vi "UHR-Fleezers Control (host) - 10.3.vi"() -> ()   [LabVIEW 2010] (continued)
        n1173 = Boolean To (0,1)(Boolean="Trap 2 ON") -> (0, 1=w4497:i16)
        n1174 = Select(t=w4497, s="Trap ON/OFF X or Y Amp?", f=w4494) -> (s? t:f=w4492:i16)
        n1175 = Select(t=w4496, s="Trap ON/OFF X or Y Amp?", f=w4494) -> (s? t:f=w4493:i16)
        n1176 = Select(t=w4495, s="Trap ON/OFF X or Y Amp?", f=w4494) -> (s? t:f=w4491:i16)
        n1177 = Select(t=w4494, s="Trap ON/OFF X or Y Amp?", f=w4497) -> (s? t:f=w4489:i16)
        n1178 = Select(t=w4494, s="Trap ON/OFF X or Y Amp?", f=w4496) -> (s? t:f=w4490:i16)
        n1179 = Select(t=w4494, s="Trap ON/OFF X or Y Amp?", f=w4495) -> (s? t:f=w4488:i16)
        n1180 = And(x="All FB On/Off", y="Feedback On/Off") -> (x .and. y?=w4486:cluster{"Set 1":bool, "Set 2":bool})
        n1181 = local read "BD 1 Amplitude 1 (%)"() -> (w4506:dbl)
        n1182 = local read "BD 1 Amplitude 2 (%)"() -> (w4505:dbl)
        n1183 = local read "BD 1 Amplitude 3 (%)"() -> (w4504:dbl)
        n1184 = Unbundle By Name(w4486) -> ("Set 1"=w4481:bool, "Set 2"=w4478:bool)
        n1185 = local read "Y RF Amplitude Limits (%)"() -> (w4474:T16)
        n1186 = local read "X RF Amplitude Limits (%)"() -> (w4475:T16)
        n1187 = local read "BD 2 Amplitude 1 (%)"() -> (w4507:dbl)
        n1188 = local read "BD 2 Amplitude 2 (%)"() -> (w4508:dbl)
        n1189 = local read "BD 2 Amplitude 3 (%)"() -> (w4509:dbl)
        n1190 = And(x="Trap 2 ON", y=w4478) -> (x .and. y?=w4476:bool)
        n1191 = And(x="Trap 1 ON", y=w4481) -> (x .and. y?=w4479:bool)
        n1192 = Multiply(x=w4493, y=w4506) -> (x*y=w4501:dbl)
        n1193 = Multiply(x=w4505, y=w4492) -> (x*y=w4499:dbl)
        n1194 = Multiply(x=w4504, y=w4491) -> (x*y=w4500:dbl)
        n1195 = Multiply(x=w4507, y=w4490) -> (x*y=w4510:dbl)
        n1196 = Multiply(x=w4508, y=w4489) -> (x*y=w4511:dbl)
        n1197 = Multiply(x=w4509, y=w4488) -> (x*y=w4512:dbl)
        n1198 = call "set RF board amplitude - interlace.vi"("Board 2 Amplitude Limits"=w4474, "Board 1 Amplitude Limits"=w4475, "error in"=w4502, "FPGA VI Reference In"=w4503, "Board 2 Amplitude 3 (%)"=w4512, "Board 1 Amplitude 3 (%)"=w4500, "Board 2 Amplitude 2 (%)"=w4511, "Board 2 Amplitude 1 (%)"=w4510, "Board 1 Amplitude 2 (%)"=w4499, "Board 1 Amplitude 1 (%)"=w4501) -> ("error out"=w4483:errorcluster, "FPGA VI Reference Out"=w4484:T19)
        n1199 = xnode "Read/Write Control"("FPGA VI Reference In"=w4484, "error in"=w4483, "FB On/Off Set 1"=w4479, "FB On/Off Set 2"=w4476) -> ("error out"=w4482:errorcluster)  [unwired: 1 out]
      }
      event "Load parameters": Value Change {
        n1200 = event-data() -> ()  [unwired: 7 out]
        n1201 = property on="Saved AOD Raster Scan Parameter Sets" class="Arr (strict)"() -> ("Index Values"=w4582:u32[])  [unwired: 2 in, 2 out]
        n1202 = Index Array(array=w4582, index=0) -> (element=w4579:u32)
        n1203 = local write "Load parameters"(FALSE ("Load parameters")) -> ()
        n1204 = Index Array(array="Saved AOD Raster Scan Parameter Sets", index=w4579) -> (element=w4578:T42)
        n1205 = Unbundle By Name(w4578) -> ("Scan Range AOD (nm) 2"=w4577:dbl, "Step Size AOD (nm) 2"=w4576:dbl, "Scan Speed AOD (nm/s) 2"=w4575:dbl, "Number of scans (AOD) 2"=w4574:u16)
        n1206 = flat-sequence {
          tunnel: w4577 -> [w4585]
          tunnel: w4576 -> [w4584]
          tunnel: w4575 -> [w4583]
          tunnel: w4574 -> [w4586]
          frame #0 {
            n1207 = local write "Scan Speed (nm/s)"(w4583) -> ()
            n1208 = local write "Scan Range (nm)"(w4585) -> ()
            n1209 = local write "Step Size (nm)"(w4584) -> ()
          }
          frame #1 {
            n1210 = property on="Number of F/B Scans (AOD)" class="DigNum (strict)"("Val(Sgnl)"=w4586) -> ()  [unwired: 2 in, 2 out]
          }
        }
      }
      event "Trap 1 (ON/OFF)", "Trap 2 (ON/OFF)": Value Change {
        n1211 = event-data() -> ()  [unwired: 7 out]
        n1212 = property on="Trap 2 ON" class="Bool (strict)"("Val(Sgnl)"="Trap 2 (ON/OFF)") -> ()  [unwired: 2 in, 2 out]
        n1213 = property on="Trap 1 ON" class="Bool (strict)"("Val(Sgnl)"="Trap 1 (ON/OFF)") -> ()  [unwired: 2 in, 2 out]
      }
      event "DIO count 1 (ticks)", "DIO count 2 (ticks)", "DIO count 3 (ticks)", "Interlace", "Number Interlace Sets", "Not-Interlacing Set": Value Change {
        n1214 = event-data() -> ()  [unwired: 7 out]
        n1215 = local read "DIO count 3 (ticks)"() -> (w4599:u32)
        n1216 = local read "DIO count 1 (ticks)"() -> (w4601:u32)
        n1217 = local read "DIO count 2 (ticks)"() -> (w4600:u32)
        n1218 = To Unsigned Byte Integer(number="Not-Interlacing Set") -> (unsigned 8bit integer=w4590:u8)
        n1219 = Add(x=w4590, y=u8 1) -> (x+y=w4594:u8)
        n1220 = xnode "Read/Write Control"("FPGA VI Reference In"=w4605, "error in"=w4603, "DIO count 1 (ticks)"=w4601, "DIO count 2 (ticks)"=w4600, "DIO count 3 (ticks)"=w4599, "Interlace ON/OFF"="Interlace", "Number Interlace Cycles"="Number Interlace Sets", "Interlace Off Parameters"=w4594) -> ("error out"=w4604:errorcluster)  [unwired: 1 out]
        n1221 = Build Array(w4601, w4600, w4599) -> (w4592:u32[])
        n1222 = Split 1D Array(array=w4592, index="Number Interlace Sets") -> (first subarray=w4602:u32[])  [unwired: 1 out]
        n1223 = Index Array(array=w4592, index=w4590) -> (element=w4591:u32)
        n1224 = Add Array Elements(numeric array=w4602) -> (sum=w4596:u32)
        n1225 = Select(t=w4596, s="Interlace", f=w4591) -> (s? t:f=→"Total Counts (ticks)":u32)
      }
      event "Reset Feedback": Value Change {
        n1226 = event-data() -> ()  [unwired: 7 out]
        n1227 = Unbundle By Name("Reset Feedback") -> ("Set 1"=w4747:bool, "Set 2"=w4746:bool)
        n1228 = xnode "Read/Write Control"("FPGA VI Reference In"=w4749, "error in"=w4744, "FB Reset Set 1"=w4747, "FB Reset Set 2"=w4746) -> ("error out"=w4745:errorcluster)  [unwired: 1 out]
      }
      event "PID Gains": Value Change {
        n1229 = event-data() -> ()  [unwired: 7 out]
        n1230 = Unbundle By Name("PID Gains") -> ("Set 1"=w4812:T14, "Set 2"=w4811:T14)
        n1231 = xnode "Read/Write Control"("FPGA VI Reference In"=w4813, "error in"=w4809, "FB Gains Set 1"=w4812, "FB Gains Set 2"=w4811) -> ("error out"=w4810:errorcluster)  [unwired: 1 out]
      }
      event "AI2 to Setpoint", "Setpoints (V)": Value Change {
        n1232 = event-data() -> ()  [unwired: 7 out]
        n1233 = xnode "Read/Write Control"("FPGA VI Reference In"=w4888, "error in"=w4884) -> ("FPGA VI Reference Out"=w4887:T19, "error out"=w4886:errorcluster, "AI2 Y Sum Set 1"=w4895:i16, "AI2 Y Sum Set 2"=w4894:i16)
        n1234 = Cluster To Array(cluster="AI2 to Setpoint") -> (array=w4898:bool[])
        n1235 = local read "AI2 (V)"() -> (w4896:cluster{"Set 1":dbl, "Set 2":dbl})
        n1236 = Or Array Elements(Boolean array=w4898) -> (logical OR=w4899:bool)
        n1237 = Bundle By Name(cluster=w4896, "Set 1"=w4895, "Set 2"=w4894) -> (w4893:cluster{"Set 1":dbl, "Set 2":dbl})
        n1238 = Divide(x=w4893, y=3276.7) -> (x/y=w4892:cluster{"Set 1":dbl, "Set 2":dbl})
        "AI2 (V)" <- w4892
        n1239 = case shown="True" w4899 {
          tunnel: [w4963 w4980] -> w4891
          tunnel: "AI2 to Setpoint" -> [_ w4976]
          tunnel: "Setpoints (V)" -> [w4964 w4979]
          tunnel: w4892 -> [_ w4973]
          frame False {
            n1240 = Multiply(x=3276.7, y=w4964) -> (x*y=w4965:cluster{"Set 1":dbl, "Set 2":dbl})
            n1241 = To Word Integer(number=w4965) -> (16bit integer=w4963:cluster{"Set 1":i16, "Set 2":i16})
          }
          frame True {
            n1242 = Unbundle By Name(w4973) -> ("Set 1"=w4972:dbl, "Set 2"=w4971:dbl)
            n1243 = Unbundle By Name(w4979) -> ("Set 1"=w4978:dbl, "Set 2"=w4977:dbl)
            n1244 = Unbundle By Name(w4976) -> ("Set 1"=w4975:bool, "Set 2"=w4974:bool)
            n1245 = Select(t=w4972, s=w4975, f=w4978) -> (s? t:f=w4970:dbl)
            n1246 = Select(t=w4971, s=w4974, f=w4977) -> (s? t:f=w4969:dbl)
            n1247 = Bundle By Name(cluster=w4979, "Set 1"=w4970, "Set 2"=w4969) -> (w4967:cluster{"Set 1":dbl, "Set 2":dbl})
            n1248 = local write "Setpoints (V)"(w4967) -> ()
            n1249 = Multiply(x=3276.7, y=w4967) -> (x*y=w4968:cluster{"Set 1":dbl, "Set 2":dbl})
            n1250 = To Word Integer(number=w4968) -> (16bit integer=w4980:cluster{"Set 1":i16, "Set 2":i16})
          }
        }
        n1251 = Unbundle By Name(w4891) -> ("Set 1"=w4890:i16, "Set 2"=w4889:i16)
        n1252 = xnode "Read/Write Control"("FPGA VI Reference In"=w4887, "error in"=w4886, "FB Setpoint Set 1"=w4890, "FB Setpoint Set 2"=w4889) -> ("error out"=w4885:errorcluster)  [unwired: 1 out]
      }
      event "Invert GI": Value Change {
        n1253 = event-data() -> ()  [unwired: 7 out]
        n1254 = xnode "Read/Write Control"("FPGA VI Reference In"=w5042, "error in"=w5040, "Invert GI"="Invert GI", "Invert GI 2"="Invert GI") -> ("error out"=w5041:errorcluster)  [unwired: 1 out]
      }
      event "Green FB Setpoint (mV)", "Green FB Gains", "Green FB On/Off", "Current When FB OFF (%)", "Green int current ON count adj": Value Change {
        n1255 = event-data() -> ()  [unwired: 7 out]
        n1256 = local read "Green FB Setpoint (mV)"() -> (w5108:dbl)
        n1257 = local read "Current When FB OFF (%)"() -> (w5111:dbl)
        n1258 = Multiply(x=w5108, y=3.2767) -> (x*y=w5107:dbl)
        n1259 = Multiply(x=w5111, y=655.35) -> (x*y=w5112:dbl)
        n1260 = To Unsigned Word Integer(number=w5112) -> (unsigned 16bit integer=w5110:u16)
        n1261 = local read "Green int current ON count adj"() -> (w5115:u32)
        n1262 = local read "Green FB Gains"() -> (w5114:T14)
        n1263 = local read "Green Laser ON/Interlacing"() -> (w5105:bool)
        n1264 = local read "Green laser mode"() -> (w5104:enum32{"Laser ON", "Laser OFF", "Interlace"})
        n1265 = local read "Green FB On/Off"() -> (w5116:bool)
        n1266 = Equal?(x=w5104, y=enum32{"Laser ON", "Laser OFF", "Interlace"}."Interlace") -> (x = y?=w5102:bool)
        n1267 = Compound Arithmetic op=AND(w5102, w5116, w5105) -> (w5106:bool)
        n1268 = xnode "Read/Write Control"("FPGA VI Reference In"=w5119, "error in"=w5118, "Green FB Setpoint"=w5107, "Green FB On/Off"=w5106, "Current Out"=w5110, "Green int current ON count adj"=w5115, "Green FB Gains"=w5114) -> ("error out"=w5117:errorcluster)  [unwired: 1 out]
      }
      event "Green laser mode", "Green Laser ON/Interlacing": Value Change {
        n1269 = event-data() -> ()  [unwired: 7 out]
        n1270 = case shown="True" "Green Laser ON/Interlacing" {
          tunnel: "Green laser mode" -> [_ w5257]
          tunnel: [enum32{"Laser ON", "Laser OFF", "Interlace"}."Laser OFF" ("Green laser mode") w5257] -> w5245
          tunnel: [FALSE w5253] -> w5244
          frame False {
          }
          frame True {
            n1271 = local read "Green FB On/Off"() -> (w5254:bool)
            n1272 = Equal?(x=w5257, y=enum32{"Laser ON", "Laser OFF", "Interlace"}."Interlace") -> (x = y?=w5255:bool)
            n1273 = And(x=w5255, y=w5254) -> (x .and. y?=w5253:bool)
          }
        }
        n1274 = xnode "Read/Write Control"("FPGA VI Reference In"=w5250, "error in"=w5248, "Operating Mode"=w5245, "Operating Mode 2"=w5245, "Green FB On/Off"=w5244) -> ("error out"=w5249:errorcluster)  [unwired: 1 out]
      }
      event "- phase (APD 1 Gate)", "+ phase (APD 1 Gate)": Value Change {
        n1275 = event-data() -> ()  [unwired: 7 out]
        n1276 = local read "Phase Adj. (APD 1 Gate)"() -> (w5336:i16)
        n1277 = Negate(x=w5336) -> (-x=w5344:i16)
        n1278 = Select(t=w5344, s="- phase (APD 1 Gate)", f=w5336) -> (s? t:f=w5343:i16)
        n1279 = Or(x="- phase (APD 1 Gate)", y="+ phase (APD 1 Gate)") -> (x .or. y?=w5339:bool)
        n1280 = xnode "Read/Write Control"("FPGA VI Reference In"=w5346, "error in"=w5345, "Phase count adjustment (APD 1 Gate)"=w5343) -> ("FPGA VI Reference Out"=w5341:T19, "error out"=w5342:errorcluster)
        n1281 = xnode "Read/Write Control"("FPGA VI Reference In"=w5341, "error in"=w5342, "+ phase (APD 1 Gate)"=w5339) -> ("error out"=w5340:errorcluster)  [unwired: 1 out]
      }
      event "+ phase (APD 2 Gate)", "- phase (APD 2 Gate)": Value Change {
        n1282 = event-data() -> ()  [unwired: 7 out]
        n1283 = local read "Phase Adj. (APD 2 Gate)"() -> (w5422:i16)
        n1284 = Negate(x=w5422) -> (-x=w5430:i16)
        n1285 = Select(t=w5430, s="- phase (APD 2 Gate)", f=w5422) -> (s? t:f=w5429:i16)
        n1286 = Or(x="- phase (APD 2 Gate)", y="+ phase (APD 2 Gate)") -> (x .or. y?=w5425:bool)
        n1287 = xnode "Read/Write Control"("FPGA VI Reference In"=w5432, "error in"=w5431, "Phase count adjustment (APD 2 Gate)"=w5429) -> ("FPGA VI Reference Out"=w5427:T19, "error out"=w5428:errorcluster)
        n1288 = xnode "Read/Write Control"("FPGA VI Reference In"=w5427, "error in"=w5428, "+ phase (APD 2 Gate)"=w5425) -> ("error out"=w5426:errorcluster)  [unwired: 1 out]
      }
      event "Phase Adj. (APD Acq)", "+ phase (APD Acq)", "- phase (APD Acq)": Value Change {
        n1289 = event-data() -> ()  [unwired: 7 out]
        n1290 = local read "Phase Adj. (APD Acq)"() -> (w5510:i16)
        n1291 = Negate(x=w5510) -> (-x=w5516:i16)
        n1292 = Select(t=w5516, s="+ phase (APD Acq)", f=w5510) -> (s? t:f=w5515:i16)
        n1293 = Or(x="+ phase (APD Acq)", y="- phase (APD Acq)") -> (x .or. y?=w5511:bool)
        n1294 = xnode "Read/Write Control"("FPGA VI Reference In"=w5518, "error in"=w5517, "Phase Count Adjustment (APD Acq)"=w5515) -> ("FPGA VI Reference Out"=w5513:T19, "error out"=w5514:errorcluster)
        n1295 = xnode "Read/Write Control"("FPGA VI Reference In"=w5513, "error in"=w5514, "+ phase (APD Acq)"=w5511) -> ("error out"=w5512:errorcluster)  [unwired: 1 out]
      }
      event "Phase adj. (GI)", "+ phase (GI)", "- phase (GI)": Value Change {
        n1296 = event-data() -> ()  [unwired: 7 out]
        n1297 = Negate(x="Phase adj. (GI)") -> (-x=w5602:i16)
        n1298 = Select(t=w5602, s="+ phase (GI)", f="Phase adj. (GI)") -> (s? t:f=w5601:i16)
        n1299 = Or(x="+ phase (GI)", y="- phase (GI)") -> (x .or. y?=w5597:bool)
        n1300 = xnode "Read/Write Control"("FPGA VI Reference In"=w5604, "error in"=w5603, "Phase count adjustment (GI)"=w5601) -> ("FPGA VI Reference Out"=w5599:T19, "error out"=w5600:errorcluster)
        n1301 = xnode "Read/Write Control"("FPGA VI Reference In"=w5599, "error in"=w5600, "+ phase (GI)"=w5597) -> ("error out"=w5598:errorcluster)  [unwired: 1 out]
      }
      event "Phase adj. (GI) 2", "+ phase (GI) 2", "- phase (GI) 2": Value Change {
        n1302 = event-data() -> ()  [unwired: 7 out]
        n1303 = Negate(x="Phase adj. (GI) 2") -> (-x=w5688:i16)
        n1304 = Select(t=w5688, s="+ phase (GI) 2", f="Phase adj. (GI) 2") -> (s? t:f=w5687:i16)
        n1305 = Or(x="+ phase (GI) 2", y="- phase (GI) 2") -> (x .or. y?=w5683:bool)
        n1306 = xnode "Read/Write Control"("FPGA VI Reference In"=w5690, "error in"=w5689, "Phase count adjustment (GI) 2"=w5687) -> ("FPGA VI Reference Out"=w5685:T19, "error out"=w5686:errorcluster)
        n1307 = xnode "Read/Write Control"("FPGA VI Reference In"=w5685, "error in"=w5686, "+ phase (GI) 2"=w5683) -> ("error out"=w5684:errorcluster)  [unwired: 1 out]
      }
      event "Phase adj. (Green FB)", "- phase (Green FB)", "+ phase (Green FB)": Value Change {
        n1308 = event-data() -> ()  [unwired: 7 out]
        n1309 = Negate(x="Phase adj. (Green FB)") -> (-x=w5774:i16)
        n1310 = Select(t=w5774, s="+ phase (Green FB)", f="Phase adj. (Green FB)") -> (s? t:f=w5773:i16)
        n1311 = Or(x="+ phase (Green FB)", y="- phase (Green FB)") -> (x .or. y?=w5769:bool)
        n1312 = xnode "Read/Write Control"("FPGA VI Reference In"=w5776, "error in"=w5775, "Phase count adjustment (Green FB)"=w5773) -> ("FPGA VI Reference Out"=w5771:T19, "error out"=w5772:errorcluster)
        n1313 = xnode "Read/Write Control"("FPGA VI Reference In"=w5771, "error in"=w5772, "+ phase (Green FB)"=w5769) -> ("error out"=w5770:errorcluster)  [unwired: 1 out]
      }
      event "Invert APD Gate", "APD Gate ON Count", "APD Gate OFF Count", "APD Gate", "APD Integration Time (s)", "APD 1 AO Mult.", "APD 2 AO Mult.": Value Change {
        n1314 = event-data() -> ()  [unwired: 7 out]
        n1315 = local read "APD Integration Time (s)"() -> (w5852:dbl)
        n1316 = local read "APD Gate ON Count"() -> (w5865:u32)
        n1317 = local read "APD Gate OFF Count"() -> (w5864:u32)
        n1318 = local read "Invert APD Gate"() -> (w5866:bool)
        n1319 = local read "APD Gate"() -> (w5863:enum32{"ON", "OFF", "Interlace"})
        n1320 = Multiply(x=w5852, y=40000000.0) -> (x*y=w5861:dbl)
        n1321 = Reciprocal(x=w5852) -> (1/x=→"APD Acq Rate (Hz)":dbl)
        n1322 = To Unsigned Long Integer(number=w5861) -> (unsigned 32bit integer=w5860:u32)
        n1323 = local read "DMA Update Period (s)"() -> (w5853:dbl)
        n1324 = Divide(x=w5853, y=w5852) -> (x/y=w5856:dbl)
        n1325 = local read "APD 1 AO Mult."() -> (w5858:i16)
        n1326 = local read "APD 2 AO Mult."() -> (w5857:i16)
        n1327 = Multiply(x=2.0, y=w5856) -> (x*y=w5855:dbl)
        n1328 = local write "APD Samples/FIFO Acq."(w5856) -> ()
        n1329 = local write "APD Elements/DMA read"(w5855) -> ()
        n1330 = xnode "Read/Write Control"("FPGA VI Reference In"=w5869, "error in"=w5868, "Invert APD Gate"=w5866, "APD Gate ON Count"=w5865, "APD Gate OFF Count"=w5864, "APD Acq Rate Count"=w5860, "APD Gate Operating Mode"=w5863, "APD 1 AO scale factor"=w5858, "APD 2 AO scale factor"=w5857) -> ("error out"=w5867:errorcluster)  [unwired: 1 out]
      }
      event "GI Frequency, ON count", "Green FB Count", "GI Frequency, OFF count": Value Change {
        n1331 = event-data() -> ()  [unwired: 7 out]
        n1332 = xnode "Read/Write Control"("FPGA VI Reference In"=w6033, "error in"=w6031, "Green interlace ON count"="GI Frequency, ON count", "Green interlace OFF count"="GI Frequency, OFF count", "Green interlace ON count 2"="GI Frequency, ON count", "Green interlace OFF count 2"="GI Frequency, OFF count", "Green FB Count"="Green FB Count") -> ("error out"=w6032:errorcluster)  [unwired: 1 out]
      }
      event "Number of F/B Scans (AOD)", "Scan Speed (nm/s)", "Scan BD", "Initial delta (MHz)", "Step Size (nm)", "Scan Range (nm)": Value Change {
        w6212 = 123.0  # AOM cal (nm/MHz)
        n1333 = event-data() -> ()  [unwired: 7 out]
        n1334 = local read "BD 1 Frequency 1 (MHz)"() -> (w6195:dbl)
        n1335 = local read "AOM X Cal (nm/MHz)"() -> (w6187:dbl)
        n1336 = local read "X RF Frequency Limits (MHz)"() -> (w6199:T16)
        n1337 = local read "Y RF Frequency Limits (MHz)"() -> (w6196:T16)
        n1338 = local read "BD 2 Frequency 1 (MHz)"() -> (w6201:dbl)
        n1339 = Negate(x="Scan Range (nm)") -> (-x=w6165:dbl)
        n1340 = Divide(x=w6165, y=w6187) -> (x/y=w6169:dbl)
        n1341 = Select(t=w6199, s="Scan BD", f=w6196) -> (s? t:f=w6198:T16)
        n1342 = Select(t=w6195, s="Scan BD", f=w6201) -> (s? t:f=w6200:dbl)
        n1343 = Unbundle By Name(w6198) -> ("Maximum"=w6207:dbl, "Minimum"=w6206:dbl)
        n1344 = Add(x=w6169, y=w6200) -> (x+y=w6204:dbl)
        n1345 = Divide(x=w6165, y="Step Size (nm)") -> (x/y=w6184:dbl)
        n1346 = Divide(x="Step Size (nm)", y=w6187) -> (x/y=w6193:dbl)
        n1347 = Absolute Value(x=w6184) -> (abs(x)=w6168:dbl)
        n1348 = Sign(1:w6165) -> (0:w6166:dbl)
        n1349 = In Range and Coerce(upper limit=w6207, x=w6204, lower limit=w6206) -> (coerced(x)=w6203:dbl, In Range?=w6205:bool)
        n1350 = To Unsigned Quad Integer(1:w6168) -> (0:w6183:u64)
        "Scan steps (AOD)" <- w6183
        n1351 = call "IR AOM freq to word.vi"("Frequency In (MHz)"=w6193) -> ("Frequency Word Out (double)"=w6190:dbl)
        n1352 = Multiply(x=w6166, y=w6190) -> (x*y=w6167:dbl)
        n1353 = Subtract(x=w6204, y=w6203) -> (x-y=w6202:dbl)
        n1354 = To Quad Integer(1:w6167) -> (0:w6189:i64)
        "Incr. int (AOD)" <- w6189
        n1355 = Subtract(x=w6169, y=w6202) -> (x-y=w6188:dbl)
        "Scan Range (MHz)" <- w6188
        n1356 = Select(t=w6169, s=w6205, f=w6188) -> (s? t:f=w6208:dbl)
        n1357 = Multiply(x=w6188, y=w6187) -> (x*y=w6186:dbl)
        n1358 = Decrement(x=w6183) -> (x-1=w6236:u64)
        n1359 = Negate(x=w6186) -> (-x=w6182:dbl)
        n1360 = local write "Scan Range (nm)"(w6182) -> ()
        n1361 = Divide(x=w6208, y=w6236) -> (x/y=w6192:dbl)
        "Scan Increment (MHz)" <- w6192
        n1362 = call "IR AOM freq to word.vi"("Frequency In (MHz)"=w6192) -> ("Frequency Word Out (double)"=w6191:dbl)
        n1363 = Divide(x="Step Size (nm)", y="Scan Speed (nm/s)") -> (x/y=w6179:dbl)
        n1364 = To Quad Integer(1:w6191) -> ()  [unwired: 1 out]
        n1365 = local read "Number Interlace Sets"() -> (w6163:u8)
        n1366 = local read "AI Count (ticks)"() -> (w6164:u32)
        n1367 = local read "Total Counts (ticks)"() -> (w6162:u32)
        n1368 = local read "# Samples/trap"() -> (w6194:u32)
        n1369 = Multiply(x=w6164, y=w6163) -> (x*y=w6161:u32)
        n1370 = Divide(x=w6162, y=w6161) -> (x/y=w6160:dbl)
        n1371 = Select(t=w6195, s="Scan BD", f=w6201) -> (s? t:f=w6233:dbl)
        "Initial freq. (MHz)" <- w6233
        n1372 = Add(x=w6208, y=w6233) -> (x+y=→"Final freq. (MHz)":dbl)
        n1373 = Divide(x=w6162, y=40000000.0) -> (x/y=w6178:dbl)
        n1374 = Divide(x=w6179, y=w6178) -> (x/y=w6177:dbl)
        n1375 = To Unsigned Quad Integer(1:w6177) -> (0:w6152:u64)
        n1376 = Quotient & Remainder(x=w6152, y=u64 2) -> (x-y*floor(x/y)=w6156:u64)  [unwired: 1 out]
        n1377 = Equal?(x=w6156, y=u64 0) -> (x = y?=w6154:bool)
        n1378 = Decrement(x=w6152) -> (x-1=w6153:u64)
        n1379 = Select(t=w6152, s=w6154, f=w6153) -> (s? t:f=w6151:u64)
        "Cycles/step (AOD)" <- w6151
        n1380 = xnode "Read/Write Control"("FPGA VI Reference In"=w6244, "error in"=w6243, "Scan steps"=w6183, "Number of scans"="Number of F/B Scans (AOD)", "Cycles per step"=w6151, "Scan freq.  increment"=w6189, "Scan BD"="Scan BD") -> ("error out"=w6242:errorcluster)  [unwired: 1 out]
        n1381 = Multiply(x=w6183, y=w6151) -> (x*y=w6237:u64)
        n1382 = Multiply(x=w6237, y=u64 2) -> (x*y=w6159:u64)
        n1383 = Multiply(x=w6160, y=w6159) -> (x*y=w6158:dbl)
        "Data points/scan (f/b)" <- w6158
        n1384 = Multiply(x=w6158, y="Number of F/B Scans (AOD)") -> (x*y=w6240:dbl)
        "Data points/scans" <- w6240
        n1385 = Divide(x=w6240, y=w6194) -> (x/y=→"N sets should be saved":dbl)
        n1386 = Multiply(x=w6237, y=w6178) -> (x*y=w6176:dbl)
        "Time/Scan (s) (AOD)" <- w6176
        n1387 = Select(t=w6208, s="Scan BD", f=0.0) -> (s? t:f=w6234:dbl)
        n1388 = Select(t=0.0, s="Scan BD", f=w6208) -> (s? t:f=w6230:dbl)
        n1389 = local read "BD 2 Frequency 2 (MHz)"() -> (w6226:dbl)
        n1390 = local read "BD 1 Frequency 2 (MHz)"() -> (w6229:dbl)
        n1391 = Add(x=w6230, y=w6201) -> (x+y=w6227:dbl)
        n1392 = Add(x=w6195, y=w6234) -> (x+y=w6228:dbl)
        n1393 = Multiply(x=w6176, y=2.0) -> (x*y=w6175:dbl)
        n1394 = Multiply(x=w6175, y="Number of F/B Scans (AOD)") -> (x*y=w6172:dbl)
        n1395 = Divide(x=w6172, y=60.0) -> (x/y=→"Time to Finish All (min)":dbl)
        n1396 = Add(x="Trap 2 Bead Size (nm)", y="Trap 1 Bead Size (nm)") -> (x+y=w6216:dbl)
        n1397 = Divide(x=w6216, y=2.0) -> (x/y=w6210:dbl)
        n1398 = local read "Initial delta (MHz)"() -> (w6213:dbl)
        n1399 = Subtract(x=w6227, y=w6226) -> (x-y=w6224:dbl)
        n1400 = Subtract(x=w6228, y=w6229) -> (x-y=w6225:dbl)
        n1401 = Square(x=w6224) -> (x^2=w6223:dbl)
        n1402 = Square(x=w6225) -> (x^2=w6222:dbl)
        n1403 = Add(x=w6222, y=w6223) -> (x+y=w6221:dbl)
        n1404 = Square Root(x=w6221) -> (sqrt(x)=w6220:dbl)
        "Final delta (MHz)" <- w6220
        n1405 = Multiply(x=w6212, y=w6220) -> (x*y=w6219:dbl)
        n1406 = Multiply(x=w6213, y=w6212) -> (x*y=w6211:dbl)
        n1407 = Subtract(x=w6211, y=w6210) -> (x-y=→"Initial sep (nm)":dbl)
        n1408 = Subtract(x=w6219, y=w6210) -> (x-y=→"Final sep (nm)":dbl)
      }
      event "Freq or Amp switch first", "Swap F1 and F2", "Freq switch delay", "Amp switch delay": Value Change {
        n1409 = event-data() -> ()  [unwired: 7 out]
        n1410 = local read "Freq or Amp switch first"() -> (w6381:bool)
        n1411 = local read "Amp switch delay"() -> (w6382:u16)
        n1412 = local read "Freq switch delay"() -> (w6384:u16)
        n1413 = local read "Swap F1 and F2"() -> (w6383:bool)
        n1414 = xnode "Read/Write Control"("FPGA VI Reference In"=w6387, "error in"=w6386, "Freq switch delay"=w6384, "Swap F1 and F2"=w6383, "Amp switch delay"=w6382, "Freq or Amp switch first"=w6381) -> ("error out"=w6385:errorcluster)  [unwired: 1 out]
      }
      event "Scan steps (MCL)", "Number of scans (MCL)", "Scan Range (V)\n(of steps)", "2D or 1D Scan", "N APD Samp/step", "Fast Scan Dir", "Continuous MCL Scanning", "Scan lines (y)": Value Change {
        w6488 = 32767.0 ("y")
        n1415 = event-data() -> ()  [unwired: 7 out]
        n1416 = Select(t="Scan lines (y)", s="2D or 1D Scan", f="Number of scans (MCL)") -> (s? t:f=w6493:u64)
        n1417 = Decrement(x="Scan steps (MCL)") -> (x-1=w6509:u64)
        n1418 = Divide(x="Scan Range (V)\n(of steps)", y=w6509) -> (x/y=w6508:dbl)
        "Desired Scan Incr (V)" <- w6508
        n1419 = local read "APD Integration Time (s)"() -> (w6501:dbl)
        n1420 = Multiply(x=w6508, y=w6488) -> (x*y=w6517:dbl)
        n1421 = Divide(x=w6517, y=10.0) -> (x/y=w6507:dbl)
        "Desired incr (int)" <- w6507
        n1422 = local read "Update Count (MCL)"() -> (w6513:u32)
        n1423 = Round Toward -Infinity(1:w6507) -> (0:w6516:dbl)
        n1424 = To Word Integer(number=w6516) -> (16bit integer=w6491:i16)
        "Actual Incr. int (MCL)" <- w6491
        n1425 = Multiply(x=w6501, y=40000000.0) -> (x*y=w6514:dbl)
        n1426 = Divide(x=w6514, y=w6513) -> (x/y=w6512:dbl)
        n1427 = Multiply(x=i16 10, y=w6491) -> (x*y=w6489:i16)
        n1428 = Multiply(x="N APD Samp/step", y=w6512) -> (x*y=w6511:dbl)
        "Cycles/step (MCL)" <- w6511
        n1429 = Divide(x=w6489, y=w6488) -> (x/y=→"Actual MCL Inc (V)":dbl)
        n1430 = Multiply(x="N APD Samp/step", y="Scan steps (MCL)") -> (x*y=w6503:dbl)
        n1431 = local read "APD Samples/FIFO Acq."() -> (w6500:dbl)
        n1432 = Multiply(x=w6503, y=u64 2) -> (x*y=w6502:dbl)
        "Data points/scan (f+b)" <- w6502
        n1433 = Multiply(x=w6502, y=w6493) -> (x*y=w6520:dbl)
        "Data points/scans (MCL)" <- w6520
        n1434 = Multiply(x=w6501, y=w6502) -> (x*y=w6494:dbl)
        "Time/f+b scan (s) (MCL)" <- w6494
        n1435 = Divide(x=w6520, y=w6500) -> (x/y=→"N sets should be saved (MCL)":dbl)
        n1436 = Multiply(x=w6494, y=w6493) -> (x*y=→"Total Time (s)":dbl)
        n1437 = Not(x="Fast Scan Dir") -> (.not. x?=w6498:bool)
        n1438 = xnode "Read/Write Control"("FPGA VI Reference In"=w6524, "error in"=w6523, "Scan steps (MCL)"="Scan steps (MCL)", "Number of scans (MCL)"=w6493, "Cycles per step (MCL)"=w6511, "Scan freq.  increment (MCL)"=w6491, "1D or 2D Scan?"="2D or 1D Scan", "MCL Scan Axis"=w6498, "Cont. Scan (MCL)"="Continuous MCL Scanning") -> ("error out"=w6522:errorcluster)  [unwired: 1 out]
      }
      event "Read Cal": Value Change {
        w6698 = 1000.0 ("y")
        n1439 = event-data() -> ()  [unwired: 7 out]
        n1440 = local read "Save file name"() -> (w6723:path)
        n1441 = local write "Read Cal"(FALSE ("Read Cal")) -> ()
        n1442 = Strip Path(path=w6723) -> (stripped path=w6722:path)  [unwired: 1 out]
        n1443 = Path To String(path=w6722) -> (string=w6721:string)
        n1444 = Concatenate Strings(w6721, "\\current.cal" ("string")) -> (w6719:string)
        n1445 = String To Path(string=w6719) -> (path=w6718:path)
        n1446 = Open/Create/Replace File(file path (use dialog)=w6718, operation (0:open)=T33."open", access (0:read/write)=enum16{"read/write", "read-only", "write-only"}."read-only") -> (refnum out=w6726:refnum<file>, error out=w6712:errorcluster)  [unwired: 1 in, 3 out]
        n1447 = Deny Access(4:w6712, 7:w6726) -> (0:w6711:errorcluster, 3:w6717:refnum<file>)  [unwired: 1 out]
        n1448 = Read from Binary File(5:0.0, 8:w6711, 9:T34."big-endian, network order" ("byte order (0:big-endian, network order)"), 10:-1 ("count (1)"), 11:w6717) -> (0:w6710:errorcluster, 2:w6708:dbl[], 3:w6713:refnum<file>)  [unwired: 2 out]
        n1449 = Array To Cluster(array=w6708) -> (cluster=w6707:T43)
        n1450 = Unbundle(w6707) -> ("[0]"=w6706:dbl, "[1]"=w6705:dbl, "[2]"=w6704:dbl, "[3]"=w6703:dbl, "[4]"=w6702:dbl, "[5]"=w6701:dbl)
        n1451 = Close File(refnum=w6713, error in=w6710) -> (error out=→"Read cal error":errorcluster)  [unwired: 1 out]
        n1452 = Multiply(x=w6701, y=w6698) -> (x*y=w6699:dbl)
        n1453 = local write "T2 kappa_x (pN/nm)"(w6703) -> ()
        n1454 = local write "T1 kappa_x (pN/nm)"(w6704) -> ()
        n1455 = local write "T1 alpha_x (nm/V)"(w6706) -> ()
        n1456 = local write "T2 alpha_x (nm/V)"(w6705) -> ()
        n1457 = Multiply(x=w6702, y=w6698) -> (x*y=w6700:dbl)
        n1458 = local write "T1 offset_x (mV)"(w6700) -> ()
        n1459 = local write "T2 offset_x (mV)"(w6699) -> ()
      }
      event "Abort MCL Scan": Value Change {
        n1460 = event-data() -> ()  [unwired: 7 out]
        n1461 = local write "MCL Scanning"(FALSE ("MCL Scanning")) -> ()
        n1462 = xnode "Read/Write Control"("FPGA VI Reference In"=w6731, "error in"=w6730, "Abort scan (MCL)"="Abort MCL Scan") -> ("error out"=w6729:errorcluster)  [unwired: 1 out]
      }
      event "Update Count (MCL)": Value Change {
        n1463 = event-data() -> ()  [unwired: 7 out]
        n1464 = xnode "Read/Write Control"("FPGA VI Reference In"=w6773, "error in"=w6772, "MCL count"="Update Count (MCL)") -> ("error out"=w6771:errorcluster)  [unwired: 1 out]
      }
      event "Phase adjust (MCL)", "+ phase (MCL)", "- phase (MCL)": Value Change {
        n1465 = event-data() -> ()  [unwired: 7 out]
        n1466 = Negate(x="Phase adjust (MCL)") -> (-x=w6819:i16)
        n1467 = Select(t=w6819, s="- phase (MCL)", f="Phase adjust (MCL)") -> (s? t:f=w6817:i16)
        n1468 = Or(x="- phase (MCL)", y="+ phase (MCL)") -> (x .or. y?=w6812:bool)
        n1469 = xnode "Read/Write Control"("FPGA VI Reference In"=w6821, "error in"=w6820, "Phase count adjustment (MCL)"=w6817) -> ("FPGA VI Reference Out"=w6813:T19, "error out"=w6814:errorcluster)
        n1470 = xnode "Read/Write Control"("FPGA VI Reference In"=w6813, "error in"=w6814, "+ phase (MCL)"=w6812) -> ("error out"=w6811:errorcluster)  [unwired: 1 out]
      }
      event "Abort AOD Scan": Value Change {
        n1471 = event-data() -> ()  [unwired: 7 out]
        n1472 = xnode "Read/Write Control"("FPGA VI Reference In"=w6900, "error in"=w6899, "Abort scan"="Abort AOD Scan") -> ("error out"=w6898:errorcluster)  [unwired: 1 out]
      }
      event "Continuous AOD Scanning": Value Change {
        n1473 = event-data() -> ()  [unwired: 7 out]
        n1474 = xnode "Read/Write Control"("FPGA VI Reference In"=w6942, "error in"=w6941, "Cont. Scan"="Continuous AOD Scanning") -> ("error out"=w6940:errorcluster)  [unwired: 1 out]
      }
      event "Index": Value Change {
        n1475 = event-data() -> ()  [unwired: 7 out]
        n1476 = call "Create new save file.vi"("Insert"="", "Ext"=".dat" ("string"), "Index In"="Index") -> ("Path Out"=→"Save file name":path, "Index Out"=w6981:dbl)
        "Save index" <- w6981
        n1477 = local write "Index"(w6981) -> ()
      }
      event "AO1", "AO2": Value Change {
        w6996 = 10.0 ("y")
        w6995 = 32767.0 ("y")
        n1478 = event-data() -> ()  [unwired: 7 out]
        n1479 = local read "AO2"() -> (w6994:dbl)
        n1480 = local read "AO1"() -> (w6991:dbl)
        n1481 = Multiply(x=w6991, y=w6995) -> (x*y=w6990:dbl)
        n1482 = Multiply(x=w6994, y=w6995) -> (x*y=w6993:dbl)
        n1483 = Divide(x=w6990, y=w6996) -> (x/y=w6989:dbl)
        n1484 = Divide(x=w6993, y=w6996) -> (x/y=w6992:dbl)
        n1485 = To Word Integer(number=w6989) -> (16bit integer=w6997:i16)
        n1486 = To Word Integer(number=w6992) -> (16bit integer=w6998:i16)
        n1487 = xnode "Read/Write Control"("FPGA VI Reference In"=w6988, "error in"=w6987, "AO1"=w6997, "AO2"=w6998) -> ("error out"=w6986:errorcluster)  [unwired: 1 out]
      }
      event "Inject Pump 1": Value Change {
        n1488 = local read "Chemyx Syringe Pump Serial Port"() -> (w7056:refnum<visa-resource-name>)
        n1489 = event-data() -> ()  [unwired: 7 out]
        n1490 = local read "Pump write delay (ms)"() -> (w7057:dbl)
        n1491 = case shown="True" "Inject Pump 1" {
          tunnel: w7057 -> [w7064 w7078]
          tunnel: w7056 -> [w7061 w7077]
          frame False {
            n1492 = flat-sequence {
              tunnel: w7061 -> [w7065]
              tunnel: [w7065] -> w7062
              tunnel: w7064 -> [_]
              tunnel: [w7068] -> w7063
              tunnel: w7062 -> [w7068]
              tunnel: w7063 -> [w7069]
              tunnel: [w7069] -> w7059
              tunnel: [w7071] -> w7060
              tunnel: w7059 -> [w7071]
              tunnel: w7060 -> [w7073]
              frame #0 {
                n1493 = call "Write to pump.vi"("string"="enter pump1", "VISA resource name"=w7065) -> ()  [unwired: 1 out]
              }
              frame #1 {
                n1494 = Wait (ms)(milliseconds to wait="Pump pause delay (ms)") -> ()  [unwired: 1 out]
              }
              frame #2 {
                n1495 = call "Write to pump.vi"("string"="stop", "VISA resource name"=w7069) -> ()  [unwired: 1 out]
              }
              frame #3 {
                n1496 = Wait (ms)(milliseconds to wait=u32 500) -> ()  [unwired: 1 out]
              }
              frame #4 {
                n1497 = call "Write to pump.vi"("string"="stop", "VISA resource name"=w7073) -> ()  [unwired: 1 out]
              }
            }
          }
          frame True {
            n1498 = flat-sequence {
              tunnel: w7077 -> [w7087]
              tunnel: w7078 -> [w7082]
              tunnel: w7078 -> [w7089]
              tunnel: w7077 -> [w7090]
              tunnel: [w7090] -> w7075
              tunnel: [w7092] -> w7076
              tunnel: w7075 -> [w7092]
              tunnel: w7076 -> [w7094]
              frame #0 {
                n1499 = local read "All Pump Parameters"() -> (w7081:T5)
                n1500 = Unbundle By Name(w7081) -> ("Pump 1"=w7088:T44)
                n1501 = call "Set pump parameters.vi"("Pump write delay (ms)"=w7082, "Volume (uL)"="Ch 2 Inject Volume (uL)", "Rate (uL/h)"="Ch 1 Inject Rate (ul/h)", "Units"=4.0, "Pump #"=1.0, "Pump Parameters In"=w7088, "VISA resource name"=w7087) -> ("Pump Parameters Out"=w7080:T44)  [unwired: 3 in]
                n1502 = Bundle By Name(cluster=w7081, "Pump 1"=w7080) -> (w7079:T5)
                n1503 = local write "All Pump Parameters"(w7079) -> ()
              }
              frame #1 {
                n1504 = Wait (ms)(milliseconds to wait=w7089) -> ()  [unwired: 1 out]
              }
              frame #2 {
                n1505 = call "Write to pump.vi"("string"="start", "VISA resource name"=w7090) -> ()  [unwired: 1 out]
              }
              frame #3 {
                n1506 = Wait (ms)(milliseconds to wait=u32 500) -> ()  [unwired: 1 out]
              }
              frame #4 {
                n1507 = call "Write to pump.vi"("string"="start", "VISA resource name"=w7094) -> ()  [unwired: 1 out]
              }
            }
          }
        }
      }
      event "Inject Pump 3": Value Change {
        n1508 = event-data() -> ()  [unwired: 7 out]
        n1509 = local read "Pump write delay (ms)"() -> (w7097:dbl)
        n1510 = case shown="False" "Inject Pump 3" {
          tunnel: w7097 -> [w7104 w7118]
          tunnel: "Chemyx Syringe Pump Serial Port" -> [w7101 w7117]
          frame False {
            n1511 = flat-sequence {
              tunnel: w7101 -> [w7105]
              tunnel: [w7105] -> w7102
              tunnel: w7104 -> [_]
              tunnel: [w7108] -> w7103
              tunnel: w7102 -> [w7108]
              tunnel: w7103 -> [w7109]
              tunnel: [w7109] -> w7099
              tunnel: [w7111] -> w7100
              tunnel: w7099 -> [w7111]
              tunnel: w7100 -> [w7113]
              frame #0 {
                n1512 = call "Write to pump.vi"("string"="enter pump3", "VISA resource name"=w7105) -> ()  [unwired: 1 out]
              }
              frame #1 {
                n1513 = local read "Pump pause delay (ms)"() -> (w7107:u32)
                n1514 = Wait (ms)(milliseconds to wait=w7107) -> ()  [unwired: 1 out]
              }
              frame #2 {
                n1515 = call "Write to pump.vi"("string"="stop", "VISA resource name"=w7109) -> ()  [unwired: 1 out]
              }
              frame #3 {
                n1516 = Wait (ms)(milliseconds to wait=u32 0) -> ()  [unwired: 1 out]
              }
              frame #4 {
                n1517 = call "Write to pump.vi"("string"="stop", "VISA resource name"=w7113) -> ()  [unwired: 1 out]
              }
            }
          }
          frame True {
            n1518 = flat-sequence {
              tunnel: w7117 -> [w7127]
              tunnel: w7118 -> [w7122]
              tunnel: w7118 -> [w7129]
              tunnel: w7117 -> [w7130]
              tunnel: [w7130] -> w7115
              tunnel: [w7133] -> w7116
              tunnel: w7115 -> [w7133]
              tunnel: w7116 -> [w7134]
              frame #0 {
                n1519 = local read "All Pump Parameters"() -> (w7121:T5)
                n1520 = Unbundle By Name(w7121) -> ("Pump 3"=w7128:T44)
                n1521 = call "Set pump parameters.vi"("Pump write delay (ms)"=w7122, "Volume (uL)"="Ch 3 Inject Volume (uL)", "Rate (uL/h)"="Ch 3 Inject Rate (ul/h)", "Units"=4.0, "Pump #"=3.0, "Pump Parameters In"=w7128, "VISA resource name"=w7127) -> ("Pump Parameters Out"=w7120:T44)  [unwired: 3 in]
                n1522 = Bundle By Name(cluster=w7121, "Pump 3"=w7120) -> (w7119:T5)
                n1523 = local write "All Pump Parameters"(w7119) -> ()
              }
              frame #1 {
                n1524 = Wait (ms)(milliseconds to wait=w7129) -> ()  [unwired: 1 out]
              }
              frame #2 {
                n1525 = call "Write to pump.vi"("string"="start", "VISA resource name"=w7130) -> ()  [unwired: 1 out]
              }
              frame #3 {
                n1526 = Wait (ms)(milliseconds to wait=u32 500) -> ()  [unwired: 1 out]
              }
              frame #4 {
                n1527 = call "Write to pump.vi"("string"="start", "VISA resource name"=w7134) -> ()  [unwired: 1 out]
              }
            }
          }
        }
      }
      event "Inject Pump 2": Value Change {
        n1528 = event-data() -> ()  [unwired: 7 out]
        n1529 = local read "Pump write delay (ms)"() -> (w7138:dbl)
        n1530 = flat-sequence {
          tunnel: w7136 -> [w7151]
          tunnel: w7138 -> [w7147]
          tunnel: "Inject Pump 2" -> [_]
          tunnel: w7138 -> [w7153]
          tunnel: w7136 -> [w7154]
          frame #0 {
            n1531 = local read "All Pump Parameters"() -> (w7146:T5)
            n1532 = Multiply(x=60.0, y="Flush Center Ch Rate (ul/m)") -> (x*y=w7143:dbl)
            n1533 = Unbundle By Name(w7146) -> ("Pump 2"=w7152:T44)
            n1534 = call "Set pump parameters.vi"("Pump write delay (ms)"=w7147, "Volume (uL)"="Flush Center Ch Volume (uL)", "Rate (uL/h)"=w7143, "Units"=3.0, "Pump #"=2.0, "Pump Parameters In"=w7152, "VISA resource name"=w7151) -> ("Pump Parameters Out"=w7145:T44)  [unwired: 3 in]
            n1535 = Bundle By Name(cluster=w7146, "Pump 2"=w7145) -> (w7144:T5)
            n1536 = local write "All Pump Parameters"(w7144) -> ()
            n1537 = Add(x="Flush Center Ch Volume (uL)", y="Total Volume\nFlushed (uL)") -> (x+y=w7140:dbl)
            n1538 = local write "Total Volume\nFlushed (uL)"(w7140) -> ()
          }
          frame #1 {
            n1539 = Wait (ms)(milliseconds to wait=w7153) -> ()  [unwired: 1 out]
          }
          frame #2 {
            n1540 = call "Write to pump.vi"("string"="start", "VISA resource name"=w7154) -> ()  [unwired: 1 out]
          }
        }
        n1541 = local read "Chemyx Syringe Pump Serial Port"() -> (w7136:refnum<visa-resource-name>)
      }
      event "Sample Channel Flow": Value Change {
        n1542 = event-data() -> ()  [unwired: 7 out]
        n1543 = Select(t="run" ("string"), s="Sample Channel Flow", f="stop" ("string")) -> (s? t:f=w7156:string)
        n1544 = Concatenate Strings(w7156, "\r") -> (w7160:string)
        n1545 = VISA Write(VISA resource name=w7162, write buffer=w7160) -> ()  [unwired: 1 in, 3 out]
      }
      event "Flip Green Filter": Value Change {
        n1546 = event-data() -> ()  [unwired: 7 out]
        n1547 = Not(x="Flip Green Filter") -> (.not. x?=w7163:bool)
        n1548 = local write "Flip Green Filter"(w7163) -> ()
        n1549 = flat-sequence {
          tunnel: w7171 -> [w7176]
          tunnel: w7170 -> [w7175]
          tunnel: [w7173] -> w7168
          tunnel: [w7172] -> w7167
          tunnel: [w7216] -> w7166
          tunnel: w7168 -> [w7216]
          tunnel: [w7215] -> w7165
          tunnel: w7167 -> [w7215]
          tunnel: w7166 -> [w7220]
          tunnel: w7165 -> [w7219]
          tunnel: [w7218] -> w7169
          frame #0 {
            n1550 = xnode "Read/Write Control"("FPGA VI Reference In"=w7176, "error in"=w7175, "Green Filter Flipper"=TRUE) -> ("FPGA VI Reference Out"=w7173:T19, "error out"=w7172:errorcluster)
          }
          frame #1 {
            n1551 = Wait (ms)(milliseconds to wait=u32 100) -> ()  [unwired: 1 out]
          }
          frame #2 {
            n1552 = xnode "Read/Write Control"("FPGA VI Reference In"=w7220, "error in"=w7219, "Green Filter Flipper"=FALSE) -> ("error out"=w7218:errorcluster)  [unwired: 1 out]
          }
        }
      }
      event "Pump 1 contents", "Pump 3 contents": Value Change {
        n1553 = event-data() -> ()  [unwired: 7 out]
        n1554 = local read "Pump 1 contents"() -> (→"Pump 1 cont disp":string)
        n1555 = local read "Pump 3 contents"() -> (→"Pump 3 cont disp":string)
      }
      event "Reset Trap Pos. FB": Value Change {
        n1556 = event-data() -> ()  [unwired: 7 out]
        n1557 = xnode "Read/Write Control"("FPGA VI Reference In"=w7264, "error in"=w7263, "Trap Pos. FB Reset"="Reset Trap Pos. FB") -> ()  [unwired: 2 out]
      }
      event "Trap Pos. FB ON": Value Change {
        n1558 = event-data() -> ()  [unwired: 7 out]
        n1559 = xnode "Read/Write Control"("FPGA VI Reference In"=w7305, "error in"=w7304, "Force feedback"="Trap Pos. FB ON") -> ()  [unwired: 2 out]
      }
      event "Trap Pos. FB Range", "Trap Pos. FB Gains", "Trap Pos. FB Mult Factor", "Trap Pos. FB Offset Factor", "Trap Pos FB Negate Action", "Trap Pos FB Monitor\nT1 or T2": Value Change {
        n1560 = event-data() -> ()  [unwired: 7 out]
        n1561 = xnode "Read/Write Control"("FPGA VI Reference In"=w7352, "error in"=w7351, "Trap Pos. FB Range"="Trap Pos. FB Range", "Trap Pos. FB Gains"="Trap Pos. FB Gains", "Trap Pos. FB Mult Factor"="Trap Pos. FB Mult Factor", "Trap Pos. FB Offset Factor"="Trap Pos. FB Offset Factor", "Trap Pos FB Negate Action"="Trap Pos FB Negate Action", "Trap Pos FB Monitor T1 or T2"="Trap Pos FB Monitor\nT1 or T2", "AI1 X Scale"="Trap Pos. AI1 X Pre-scale") -> ()  [unwired: 2 out]
      }
      event "Trap Pos FB SP": Value Change {
        n1562 = event-data() -> ()  [unwired: 7 out]
        n1563 = xnode "Read/Write Control"("FPGA VI Reference In"=w7540, "error in"=w7539, "Trap Pos. FB SP"="Trap Pos FB SP") -> ()  [unwired: 2 out]
      }
      event "Set SP to Reading": Value Change {
        n1564 = event-data() -> ()  [unwired: 7 out]
        n1565 = local read "Trap Pos FB Monitor\nT1 or T2"() -> (w7593:bool)
        n1566 = local read "Trap X AI1 (DMA)"() -> (w7596:T13)
        n1567 = local read "Trap X (AI1)"() -> (w7599:T10)
        n1568 = Unbundle By Name(w7599) -> ("Trap 1"=w7598:fxp<+/-,16,1>, "Trap 2"=w7597:fxp<+/-,16,1>)
        n1569 = Unbundle By Name(w7596) -> ("Set 1"=w7595:fxp<+/-,16,1>, "Set 2"=w7594:fxp<+/-,16,1>)
        n1570 = Select(t=w7598, s=w7593, f=w7597) -> (s? t:f=w7592:fxp<+/-,16,1>)
        n1571 = Select(t=w7595, s=w7593, f=w7594) -> (s? t:f=w7591:fxp<+/-,16,1>)
        n1572 = Not(x="Set SP Using...") -> (.not. x?=w7586:bool)
        n1573 = Select(t=w7592, s=w7586, f=w7591) -> (s? t:f=w7587:fxp<+/-,16,1>)
        n1574 = xnode "Read/Write Control"("FPGA VI Reference In"=w7589, "error in"=w7588, "Trap Pos. FB SP"=w7587) -> ()  [unwired: 2 out]
        n1575 = local write "Trap Pos FB SP"(w7587) -> ()
      }
      event "Trap Pos. FB Out Scale 2^n": Value Change {
        n1576 = event-data() -> ()  [unwired: 7 out]
        n1577 = Scale By Power Of 2(n="Trap Pos. FB Out Scale 2^n", x=ext 1.0) -> (x*2^n=w7646:ext)
        n1578 = property on="Trap Pos. FB Mult Factor" class="DigNum (strict)"("Val(Sgnl)"=w7646) -> ()  [unwired: 2 in, 2 out]
      }
      event "Trap Pos FB Int Count": Value Change {
        n1579 = event-data() -> ()  [unwired: 7 out]
        n1580 = xnode "Read/Write Control"("FPGA VI Reference In"=w7651, "error in"=w7650, "Trap Pos FB Int Count"="Trap Pos FB Int Count") -> ()  [unwired: 2 out]
      }
    }
    "error out 2" <- w4179
    n1581 = node-c288() -> ()  [unwired: 2 out]
  }
  n1582 = timed-loop "Run Scripts, including: stage motion" {
    tunnel: w41 -> [w7691]
    tunnel: w40 -> [w7692]
    tunnel: [w7692] -> w39
    tunnel: [w7691] -> w38
    timing: w37 -> [_]
    timing-out: [_] -> w36
    tunnel: w22 -> [w7690]
    tunnel: w23 -> [w7689]
    stop <- w7693 stop-if-true
    n1583 = node-c288() -> ()  [unwired: 1 in, 1 out]
    n1584 = event shown="[3] \"Move Cap. 2 (ADig Left)\": Value Change" {
      selector: _ -> [_ _ _ _ _ _ _ _ _ _ _ _ _ _ _ _]
      dyn-events: _ -> [_ _ _ _ _ _ _ _ _ _ _ _ _ _ _ _]
      timeout: _ -> [_ _ _ _ _ _ _ _ _ _ _ _ _ _ _ _]
      tunnel: ["Set Position" "Move to Position" "Move Cap. 1 (DNA Right)" "Move Cap. 2 (ADig Left)" _ "Cal/Data Acq. Spot" "Dump Beads" "Dip for Protein" _ _ "Got ADig bead" "Got DNA bead" "Take Stepping Data" _ "Take Detection Laser\nImage" _] -> _
      tunnel: [_ _ _ _ _ _ _ _ _ _ _ _ _ _ _ w8184] -> w7693
      tunnel: w7691 -> [w7711 w7719 w7743 w7798 w7843 w7879 w7957 w7982 w8032 w8058 _ _ _ _ _ _]
      tunnel: w7692 -> [w7712 w7720 w7744 w7799 w7844 w7880 w7958 w7983 w8033 w8059 _ _ _ _ _ _]
      tunnel: w7690 -> [_ _ w7741 w7795 _ _ _ _ _ _ _ _ _ _ _ _]
      tunnel: w7689 -> [_ _ w7740 w7796 _ _ _ _ _ _ _ _ _ _ _ _]
      event "Set Position", "Set Position 2", "Set Position 3", "Set Position 4", "Set Position 5", "Set Position 1": Value Change {
        n1585 = event-data() -> ()  [unwired: 1 in, 5 out]
        n1586 = Build Array("Set Position 1", "Set Position 2", "Set Position 3", "Set Position 4", "Set Position 5") -> (w7710:bool[])
        n1587 = Boolean Array To Number(Boolean array=w7710) -> (number=w7709:u32)
        n1588 = Logarithm Base 2(1:w7709) -> (0:w7701:dbl)
        n1589 = call "Read Stage Position.vi"("error in"=w7711, "VISA resource name in"=w7712) -> ("Current Position"=w7716:cluster{dbl, dbl, dbl}, "error out"=w7715:errorcluster)  [unwired: 2 out]
        n1590 = Decrement(x="Position") -> (x-1=w7699:dbl)
        n1591 = Greater Or Equal?(x=w7701, y=0.0) -> (x >= y?=w7702:bool)
        n1592 = local write "Stage Control Serial Error"(w7715) -> ()
        n1593 = Cluster To Array(cluster=w7716) -> (array=w7713:dbl[])
        n1594 = Select(t=w7701, s=w7702, f=w7699) -> (s? t:f=w7698:dbl)
        n1595 = Increment(x=w7698) -> (x+1=w7697:dbl)
        n1596 = Build Array (concatenate)(w7697, w7713) -> (w7696:dbl[])
        n1597 = Replace Array Subset(array="Saved Stage Positions", new element=w7696, index (row)=w7698) -> (w7714:dbl[][])  [unwired: 1 in]
        n1598 = local write "Saved Stage Positions"(w7714) -> ()
      }
      event "Move to Position": Value Change {
        n1599 = event-data() -> ()  [unwired: 1 in, 5 out]
        n1600 = flat-sequence {
          tunnel: w7720 -> [w7723]
          tunnel: w7719 -> [w7722]
          frame #0 {
            n1601 = local read "Position"() -> (w7735:dbl)
            n1602 = local read "Saved Stage Positions"() -> (w7733:dbl[][])
            n1603 = Decrement(x=w7735) -> (x-1=w7732:dbl)
            n1604 = Array Subset(array=w7733, index (row)=w7732, length (row)=1 ("length"), index (col)=1 ("index"), length (col)=3 ("length")) -> (w7729:dbl[][])
            n1605 = Reshape Array(w7729, 3 ("dimension size")) -> (w7727:dbl[])
            n1606 = Array To Cluster(array=w7727) -> (cluster=w7726:cluster{"[0]":dbl, "[1]":dbl, "[2]":dbl})
            n1607 = call "Set Stage Position.vi"("Position"=w7726, "error in"=w7722, "VISA resource name in"=w7723) -> ("error out"=w7725:errorcluster)  [unwired: 2 out]
            n1608 = local write "Stage Control Serial Error"(w7725) -> ()
            n1609 = local write "Stage Moving"(TRUE ("Stage Moving")) -> ()
          }
          frame #1 {
            n1610 = call <vilib>:"Beep.vi"() -> ()  [unwired: 3 in, 9 out]
            n1611 = local write "Stage Moving"(FALSE ("Stage Moving")) -> ()
          }
        }
      }
      event "Move Cap. 1 (DNA Right)": Value Change {
        n1612 = event-data() -> ()  [unwired: 1 in, 5 out]
        n1613 = local write "Move Cap. 1 (DNA Right)"(FALSE ("Move Cap. 1 (DNA Right)")) -> ()
        n1614 = flat-sequence {
          tunnel: w7744 -> [w7752]